vi "Dresden R2R Sputter 03.02.2018 IY24.vi"() -> ()   [LabVIEW 2009] (continued)
                                n21135 = local write "Semi"(TRUE ("Semi")) -> ()
                                }
                                }
                                n21136 = local read "Ch4_Air_press_di"() -> (w22217:bool)
                                n21137 = case shown="True" w22217 {
                                tunnel: [TRUE FALSE] -> w22220
                                frame #0 {
                                }
                                frame #1 {
                                n21138 = Wait Until Next ms Multiple(millisecond multiple=u32 200) -> ()  [unwired: 1 out]
                                }
                                }
                                n21139 = local read "Semi"() -> (w22219:bool)
                                n21140 = Or(x=w22220, y=w22219) -> (x .or. y?=w22218:bool)
                                }
                              }
                              frame #1 {
                              }
                            }
                          }
                          frame #1 {
                            n21141 = local read "Semi"() -> (w22228:bool)
                            n21142 = case shown="False" w22228 {
                              frame #0 {
                                n21143 = Wait Until Next ms Multiple(millisecond multiple=u32 1000) -> ()  [unwired: 1 out]
                                n21144 = local write "Ch4_PV0"(TRUE ("PA0")) -> ()
                                n21145 = local write "Ch4_PA0"(TRUE ("PA0")) -> ()
                              }
                              frame #1 {
                              }
                            }
                          }
                        }
                      }
                      frame #1 {
                      }
                    }
                  }
                  frame #2 {
                    n21146 = local read "Semi"() -> (w22232:bool)
                    n21147 = case shown="False" w22232 {
                      frame #0 {
                        n21148 = stacked-sequence {
                          frame #0 {
                            n21149 = local read "Semi"() -> (w22233:bool)
                            n21150 = case shown="False" w22233 {
                              frame #0 {
                                n21151 = while {
                                i -> [w22240]
                                stop <- w22236 stop-if-true
                                n21152 = Greater?(x=w22240, y=50) -> (0:w22234:bool)
                                n21153 = case shown="True" w22234 {
                                frame #0 {
                                }
                                frame #1 {
                                n21154 = local write "Error Message"("Start up process cancelled because\nchamber door is open.\nPlease close the door." ("Error Message")) -> ()
                                n21155 = local write "Semi"(TRUE ("Semi")) -> ()
                                }
                                }
                                n21156 = local read "Ch4_Ds_di"() -> (w22235:bool)
                                n21157 = case shown="False" w22235 {
                                tunnel: [TRUE FALSE] -> w22238
                                frame #0 {
                                }
                                frame #1 {
                                n21158 = Wait Until Next ms Multiple(millisecond multiple=u32 200) -> ()  [unwired: 1 out]
                                }
                                }
                                n21159 = local read "Semi"() -> (w22237:bool)
                                n21160 = Or(x=w22238, y=w22237) -> (x .or. y?=w22236:bool)
                                }
                              }
                              frame #1 {
                              }
                            }
                          }
                          frame #1 {
                            n21161 = local read "Semi"() -> (w22246:bool)
                            n21162 = case shown="False" w22246 {
                              frame #0 {
                                n21163 = local write "Ch4_PV1"(TRUE ("PA0")) -> ()
                                n21164 = local write "Ch4_PA1"(TRUE ("PA0")) -> ()
                                n21165 = Wait Until Next ms Multiple(millisecond multiple=u32 1000) -> ()  [unwired: 1 out]
                              }
                              frame #1 {
                              }
                            }
                          }
                        }
                      }
                      frame #1 {
                      }
                    }
                  }
                  frame #3 {
                    n21166 = local read "Semi"() -> (w22250:bool)
                    n21167 = case shown="False" w22250 {
                      frame #0 {
                        n21168 = stacked-sequence {
                          frame #0 {
                            n21169 = local read "Semi"() -> (w22251:bool)
                            n21170 = case shown="False" w22251 {
                              frame #0 {
                                n21171 = while {
                                i -> [w22258]
                                stop <- w22254 stop-if-true
                                n21172 = Greater?(x=w22258, y=50) -> (0:w22252:bool)
                                n21173 = case shown="True" w22252 {
                                frame #0 {
                                }
                                frame #1 {
                                n21174 = local write "Error Message"("Start up process cancelled because\nsystem water flow is not enough.\nPlease check main water flow connections." ("Error Message")) -> ()
                                n21175 = local write "Semi"(TRUE ("Semi")) -> ()
                                }
                                }
                                n21176 = local read "Cnt_wfs_di"() -> (w22253:bool)
                                n21177 = case shown="False" w22253 {
                                tunnel: [TRUE FALSE] -> w22256
                                frame #0 {
                                }
                                frame #1 {
                                n21178 = Wait Until Next ms Multiple(millisecond multiple=u32 200) -> ()  [unwired: 1 out]
                                }
                                }
                                n21179 = local read "Semi"() -> (w22255:bool)
                                n21180 = Or(x=w22256, y=w22255) -> (x .or. y?=w22254:bool)
                                }
                              }
                              frame #1 {
                              }
                            }
                          }
                          frame #1 {
                            n21181 = local read "Semi"() -> (w22264:bool)
                            n21182 = case shown="False" w22264 {
                              frame #0 {
                                n21183 = Wait Until Next ms Multiple(millisecond multiple=u32 1000) -> ()  [unwired: 1 out]
                                n21184 = local write "Ch4_PA2"(TRUE ("PA0")) -> ()
                                n21185 = local write "Ch4_PV2"(TRUE ("PA0")) -> ()
                              }
                              frame #1 {
                              }
                            }
                          }
                        }
                      }
                      frame #1 {
                      }
                    }
                  }
                  frame #4 {
                    n21186 = local read "Semi"() -> (w22268:bool)
                    n21187 = case shown="False" w22268 {
                      frame #0 {
                        n21188 = disable-structure shown="Disabled" {
                          frame #0 {
                            n21189 = stacked-sequence {
                              frame #0 {
                                n21190 = local read "Semi"() -> (w22269:bool)
                                n21191 = case shown="False" w22269 {
                                frame #0 {
                                n21192 = local write "Ch4_WFC_do"(TRUE ("Ch1_WFC_do")) -> ()
                                }
                                frame #1 {
                                }
                                }
                              }
                              frame #1 {
                                n21193 = local read "Semi"() -> (w22271:bool)
                                n21194 = case shown="False" w22271 {
                                frame #0 {
                                n21195 = while {
                                i -> [w22278]
                                stop <- w22274 stop-if-true
                                n21196 = Greater?(x=w22278, y=50) -> (0:w22272:bool)
                                n21197 = case shown="True" w22272 {
                                frame #0 {
                                }
                                frame #1 {
                                n21198 = local write "Error Message"("Start up process cancelled because\nchamber water flow is not enough.\nPlease check chamber water \nflow connections." ("Error Message")) -> ()
                                n21199 = local write "Semi"(TRUE ("Semi")) -> ()
                                }
                                }
                                n21200 = local read "Ch4_WFS_di"() -> (w22273:bool)
                                n21201 = case shown="False" w22273 {
                                tunnel: [TRUE FALSE] -> w22276
                                frame #0 {
                                }
                                frame #1 {
                                n21202 = Wait Until Next ms Multiple(millisecond multiple=u32 200) -> ()  [unwired: 1 out]
                                n21203 = local write "Ch4_WFC_do"(TRUE ("Ch1_WFC_do")) -> ()
                                }
                                }
                                n21204 = local read "Semi"() -> (w22275:bool)
                                n21205 = Or(x=w22276, y=w22275) -> (x .or. y?=w22274:bool)
                                }
                                }
                                frame #1 {
                                }
                                }
                              }
                              frame #2 {
                                n21206 = local read "Semi"() -> (w22285:bool)
                                n21207 = case shown="False" w22285 {
                                frame #0 {
                                n21208 = Wait Until Next ms Multiple(millisecond multiple=u32 1000) -> ()  [unwired: 1 out]
                                }
                                frame #1 {
                                }
                                }
                              }
                            }
                          }
                          frame #1 {
                          }
                        }
                      }
                      frame #1 {
                      }
                    }
                  }
                  frame #5 {
                    n21209 = local read "Semi"() -> (w22287:bool)
                    n21210 = case shown="False" w22287 {
                      frame #0 {
                        n21211 = stacked-sequence {
                          frame #0 {
                            n21212 = local read "Semi"() -> (w22288:bool)
                            n21213 = case shown="False" w22288 {
                              frame #0 {
                                n21214 = local write "Ch3_Trns_gv_close_do"(TRUE ("Ch1_WFC_do")) -> ()
                              }
                              frame #1 {
                              }
                            }
                          }
                          frame #1 {
                            n21215 = local read "Semi"() -> (w22290:bool)
                            n21216 = case shown="False" w22290 {
                              frame #0 {
                                n21217 = while {
                                i -> [w22297]
                                stop <- w22293 stop-if-true
                                n21218 = Greater?(x=w22297, y=300) -> (0:w22291:bool)
                                n21219 = case shown="True" w22291 {
                                frame #0 {
                                }
                                frame #1 {
                                n21220 = local write "Error Message"("Start up process cancelled because\nchamber Trns GV between \nCH3 and CH4 not closed.\nPlease check  GV connection." ("Error Message")) -> ()
                                n21221 = local write "Semi"(TRUE ("Semi")) -> ()
                                }
                                }
                                n21222 = local read "Ch3_Trns_gv_close_di"() -> (w22292:bool)
                                n21223 = case shown="False" w22292 {
                                tunnel: [TRUE FALSE] -> w22295
                                frame #0 {
                                }
                                frame #1 {
                                n21224 = Wait Until Next ms Multiple(millisecond multiple=u32 200) -> ()  [unwired: 1 out]
                                n21225 = local write "Ch3_Trns_gv_open_do"(FALSE ("Ch1_Trns_gv_open_do")) -> ()
                                n21226 = local write "Ch3_Trns_gv_close_do"(TRUE ("Ch1_Trns_gv_close_do")) -> ()
                                }
                                }
                                n21227 = local read "Semi"() -> (w22294:bool)
                                n21228 = Or(x=w22295, y=w22294) -> (x .or. y?=w22293:bool)
                                }
                              }
                              frame #1 {
                              }
                            }
                          }
                          frame #2 {
                            n21229 = local read "Semi"() -> (w22305:bool)
                            n21230 = case shown="False" w22305 {
                              frame #0 {
                                w22306 = TRUE ("PA0")
                                n21231 = Wait Until Next ms Multiple(millisecond multiple=u32 1000) -> ()  [unwired: 1 out]
                                n21232 = local write "Ch4_PA4"(w22306) -> ()
                                n21233 = local write "Ch4_PV4"(w22306) -> ()
                              }
                              frame #1 {
                              }
                            }
                          }
                        }
                      }
                      frame #1 {
                      }
                    }
                  }
                }
              }
              frame #1 {
              }
            }
          }
          frame #1 {
            # "ROUTINE CHECK"
            n21234 = local read "Semi"() -> (w22308:bool)
            n21235 = case shown="False" w22308 {
              frame #0 {
                n21236 = local read "Ch4_pressure2"() -> (w22310:dbl)
                n21237 = Greater Or Equal?(x=w22310, y=0.9) -> (x >= y?=w22309:bool)
                n21238 = case shown="True" w22309 {
                  frame #0 {
                    # "PUMPING CH1 LOWER THAN 0.9 TORR"
                    n21239 = local read "Semi"() -> (w22312:bool)
                    n21240 = case shown="False" w22312 {
                      frame #0 {
                        n21241 = stacked-sequence {
                          frame #0 {
                            # "Close CH-VBV"
                            n21242 = local read "Semi"() -> (w22313:bool)
                            n21243 = case shown="False" w22313 {
                              frame #0 {
                                n21244 = stacked-sequence {
                                frame #0 {
                                n21245 = local read "Semi"() -> (w22314:bool)
                                n21246 = case shown="False" w22314 {
                                frame #0 {
                                n21247 = while {
                                i -> [w22321]
                                stop <- w22315 stop-if-true
                                n21248 = Greater?(x=w22321, y=50) -> (0:w22319:bool)
                                n21249 = case shown="True" w22319 {
                                frame #0 {
                                }
                                frame #1 {
                                n21250 = local write "Semi"(TRUE ("Semi")) -> ()
                                n21251 = local write "Error Message"("Start up process  cancelled\nbecause  CH-VBV not closed.\nPlease check  CH4-VBV connections." ("Error Message")) -> ()
                                }
                                }
                                n21252 = local read "Ch4_Ch_vbv_di"() -> (w22318:bool)
                                n21253 = case shown="True" w22318 {
                                tunnel: [TRUE FALSE] -> w22317
                                frame #0 {
                                }
                                frame #1 {
                                n21254 = Wait Until Next ms Multiple(millisecond multiple=u32 200) -> ()  [unwired: 1 out]
                                n21255 = local write "Ch4_Ch_vbv_do"(FALSE ("Ch1_Tp_bv_do")) -> ()
                                }
                                }
                                n21256 = local read "Semi"() -> (w22316:bool)
                                n21257 = Or(x=w22317, y=w22316) -> (x .or. y?=w22315:bool)
                                }
                                }
                                frame #1 {
                                }
                                }
                                }
                                frame #1 {
                                n21258 = local read "Semi"() -> (w22328:bool)
                                n21259 = case shown="False" w22328 {
                                frame #0 {
                                n21260 = local write "Ch4_PV5"(TRUE ("Pd5")) -> ()
                                n21261 = Wait Until Next ms Multiple(millisecond multiple=u32 1000) -> ()  [unwired: 1 out]
                                }
                                frame #1 {
                                }
                                }
                                }
                                }
                              }
                              frame #1 {
                              }
                            }
                          }
                          frame #1 {
                            # "Close PL-VBV"
                            n21262 = local read "Semi"() -> (w22331:bool)
                            n21263 = case shown="False" w22331 {
                              frame #0 {
                                n21264 = stacked-sequence {
                                frame #0 {
                                n21265 = local read "Semi"() -> (w22332:bool)
                                n21266 = case shown="False" w22332 {
                                frame #0 {
                                n21267 = while {
                                i -> [w22339]
                                stop <- w22333 stop-if-true
                                n21268 = Greater?(x=w22339, y=50) -> (0:w22337:bool)
                                n21269 = case shown="True" w22337 {
                                frame #0 {
                                }
                                frame #1 {
                                n21270 = local write "Semi"(TRUE ("Semi")) -> ()
                                n21271 = local write "Error Message"("Start up process  cancelled\nbecause  PL-VBV not closed.\nPlease check PL4-VBV connections." ("Error Message")) -> ()
                                }
                                }
                                n21272 = local read "Ch4_Pl_vbv_di"() -> (w22336:bool)
                                n21273 = case shown="True" w22336 {
                                tunnel: [TRUE FALSE] -> w22335
                                frame #0 {
                                }
                                frame #1 {
                                n21274 = Wait Until Next ms Multiple(millisecond multiple=u32 200) -> ()  [unwired: 1 out]
                                n21275 = local write "Ch4_Pl_vbv_do"(FALSE ("Ch1_Tp_bv_do")) -> ()
                                }
                                }
                                n21276 = local read "Semi"() -> (w22334:bool)
                                n21277 = Or(x=w22335, y=w22334) -> (x .or. y?=w22333:bool)
                                }
                                }
                                frame #1 {
                                }
                                }
                                }
                                frame #1 {
                                n21278 = local read "Semi"() -> (w22346:bool)
                                n21279 = case shown="False" w22346 {
                                frame #0 {
                                n21280 = local write "Ch4_PV6"(TRUE ("P03")) -> ()
                                n21281 = Wait Until Next ms Multiple(millisecond multiple=u32 1000) -> ()  [unwired: 1 out]
                                }
                                frame #1 {
                                }
                                }
                                }
                                }
                              }
                              frame #1 {
                              }
                            }
                          }
                          frame #2 {
                            # "Close CH-ATM"
                            n21282 = local read "Semi"() -> (w22349:bool)
                            n21283 = case shown="False" w22349 {
                              frame #0 {
                                n21284 = stacked-sequence {
                                frame #0 {
                                n21285 = local read "Semi"() -> (w22350:bool)
                                n21286 = case shown="False" w22350 {
                                frame #0 {
                                n21287 = while {
                                i -> [w22357]
                                stop <- w22351 stop-if-true
                                n21288 = Greater?(x=w22357, y=50) -> (0:w22355:bool)
                                n21289 = case shown="True" w22355 {
                                frame #0 {
                                }
                                frame #1 {
                                n21290 = local write "Semi"(TRUE ("Semi")) -> ()
                                n21291 = local write "Error Message"("Start up process  cancelled\nbecause CH-ATM not closed.\nPlease check CH4-ATM connections." ("Error Message")) -> ()
                                }
                                }
                                n21292 = local read "Ch4_Ch_atm_di"() -> (w22354:bool)
                                n21293 = case shown="True" w22354 {
                                tunnel: [TRUE FALSE] -> w22353
                                frame #0 {
                                }
                                frame #1 {
                                n21294 = Wait Until Next ms Multiple(millisecond multiple=u32 200) -> ()  [unwired: 1 out]
                                n21295 = local write "Ch4_Ch_atm_do"(TRUE ("Ch1_Tp_bv_do")) -> ()
                                }
                                }
                                n21296 = local read "Semi"() -> (w22352:bool)
                                n21297 = Or(x=w22353, y=w22352) -> (x .or. y?=w22351:bool)
                                }
                                }
                                frame #1 {
                                }
                                }
                                }
                                frame #1 {
                                n21298 = local read "Semi"() -> (w22364:bool)
                                n21299 = case shown="False" w22364 {
                                frame #0 {
                                n21300 = Wait Until Next ms Multiple(millisecond multiple=u32 1000) -> ()  [unwired: 1 out]
                                n21301 = local write "Ch4_PV7"(TRUE ("P03")) -> ()
                                }
                                frame #1 {
                                }
                                }
                                }
                                }
                              }
                              frame #1 {
                              }
                            }
                          }
                          frame #3 {
                            # "Close PL-ATM"
                            n21302 = local read "Semi"() -> (w22367:bool)
                            n21303 = case shown="False" w22367 {
                              frame #0 {
                                n21304 = stacked-sequence {
                                frame #0 {
                                n21305 = local read "Semi"() -> (w22368:bool)
                                n21306 = case shown="False" w22368 {
                                frame #0 {
                                n21307 = while {
                                i -> [w22375]
                                stop <- w22369 stop-if-true
                                n21308 = Greater?(x=w22375, y=50) -> (0:w22373:bool)
                                n21309 = case shown="True" w22373 {
                                frame #0 {
                                }
                                frame #1 {
                                n21310 = local write "Semi"(TRUE ("Semi")) -> ()
                                n21311 = local write "Error Message"("Start up process  cancelled\nbecause PL-ATM not closed.\nPlease check PL4-ATM connections." ("Error Message")) -> ()
                                }
                                }
                                n21312 = local read "Ch4_Pl_atm_di"() -> (w22372:bool)
                                n21313 = case shown="True" w22372 {
                                tunnel: [TRUE FALSE] -> w22371
                                frame #0 {
                                }
                                frame #1 {
                                n21314 = Wait Until Next ms Multiple(millisecond multiple=u32 200) -> ()  [unwired: 1 out]
                                n21315 = local write "Ch4_Pl_atm_do"(TRUE ("Ch1_Tp_bv_do")) -> ()
                                }
                                }
                                n21316 = local read "Semi"() -> (w22370:bool)
                                n21317 = Or(x=w22371, y=w22370) -> (x .or. y?=w22369:bool)
                                }
                                }
                                frame #1 {
                                }
                                }
                                }
                                frame #1 {
                                n21318 = local read "Semi"() -> (w22382:bool)
                                n21319 = case shown="False" w22382 {
                                frame #0 {
                                n21320 = Wait Until Next ms Multiple(millisecond multiple=u32 1000) -> ()  [unwired: 1 out]
                                n21321 = local write "Ch4_PV8"(TRUE ("P03")) -> ()
                                }
                                frame #1 {
                                }
                                }
                                }
                                }
                              }
                              frame #1 {
                              }
                            }
                          }
                          frame #4 {
                            # "START MP"
                            n21322 = local read "Semi"() -> (w22385:bool)
                            n21323 = case shown="False" w22385 {
                              frame #0 {
                                n21324 = stacked-sequence {
                                frame #0 {
                                n21325 = local read "Semi"() -> (w22386:bool)
                                n21326 = case shown="False" w22386 {
                                frame #0 {
                                n21327 = while {
                                i -> [w22393]
                                stop <- w22387 stop-if-true
                                n21328 = Greater?(x=w22393, y=50) -> (0:w22391:bool)
                                n21329 = case shown="True" w22391 {
                                frame #0 {
                                }
                                frame #1 {
                                n21330 = local write "Semi"(TRUE ("Semi")) -> ()
                                n21331 = local write "Error Message"("Start up process  cancelled\nbecause MP4 not started.\nPlease check MP4 connections." ("Error Message")) -> ()
                                }
                                }
                                n21332 = local read "Ch4_Mp_di"() -> (w22390:bool)
                                n21333 = case shown="False" w22390 {
                                tunnel: [FALSE TRUE] -> w22389
                                frame #0 {
                                n21334 = Wait Until Next ms Multiple(millisecond multiple=u32 200) -> ()  [unwired: 1 out]
                                n21335 = local write "Ch4_Mp_do"(TRUE ("Ch1_Tp_bv_do")) -> ()
                                }
                                frame #1 {
                                }
                                }
                                n21336 = local read "Semi"() -> (w22388:bool)
                                n21337 = Or(x=w22389, y=w22388) -> (x .or. y?=w22387:bool)
                                }
                                }
                                frame #1 {
                                }
                                }
                                }
                                frame #1 {
                                n21338 = local read "Semi"() -> (w22400:bool)
                                n21339 = case shown="False" w22400 {
                                frame #0 {
                                n21340 = local write "Ch4_PV9"(TRUE ("P03")) -> ()
                                n21341 = Wait Until Next ms Multiple(millisecond multiple=u32 1000) -> ()  [unwired: 1 out]
                                }
                                frame #1 {
                                }
                                }
                                }
                                }
                              }
                              frame #1 {
                              }
                            }
                          }
                          frame #5 {
                            # "CHECK PL-PRESSURE"
                            n21342 = local read "Semi"() -> (w22403:bool)
                            n21343 = case shown="False" w22403 {
                              frame #0 {
                                n21344 = stacked-sequence {
                                frame #0 {
                                n21345 = local read "Semi"() -> (w22404:bool)
                                n21346 = case shown="False" w22404 {
                                frame #0 {
                                n21347 = while {
                                i -> [w22413]
                                stop <- w22408 stop-if-true
                                n21348 = Greater?(x=w22413, y=240) -> (0:w22411:bool)
                                n21349 = case shown="True" w22411 {
                                frame #0 {
                                }
                                frame #1 {
                                n21350 = local write "Semi"(TRUE ("Semi")) -> ()
                                n21351 = local write "Error Message"("Start up process was cancelled.\nPlease check Pipeline \nvacuum connections." ("Error Message")) -> ()
                                }
                                }
                                n21352 = local read "Pl_pg_press_ch4"() -> (w22407:dbl)
                                n21353 = Less?(x=w22407, y=0.9) -> (x < y?=w22405:bool)
                                n21354 = case shown="False" w22405 {
                                tunnel: [FALSE TRUE] -> w22410
                                frame #0 {
                                n21355 = Wait Until Next ms Multiple(millisecond multiple=u32 200) -> ()  [unwired: 1 out]
                                }
                                frame #1 {
                                }
                                }
                                n21356 = local read "Semi"() -> (w22409:bool)
                                n21357 = Or(x=w22410, y=w22409) -> (x .or. y?=w22408:bool)
                                }
                                }
                                frame #1 {
                                }
                                }
                                }
                                frame #1 {
                                n21358 = local read "Semi"() -> (w22419:bool)
                                n21359 = case shown="False" w22419 {
                                frame #0 {
                                n21360 = Wait Until Next ms Multiple(millisecond multiple=u32 1000) -> ()  [unwired: 1 out]
                                n21361 = local write "Ch4_PV10"(TRUE ("P03")) -> ()
                                }
                                frame #1 {
                                }
                                }
                                }
                                }
                              }
                              frame #1 {
                              }
                            }
                          }
                          frame #6 {
                            # "CHECK CH-PRESSURE"
                            n21362 = local read "Semi"() -> (w22422:bool)
                            n21363 = case shown="False" w22422 {
                              frame #0 {
                                n21364 = stacked-sequence {
                                frame #0 {
                                n21365 = local read "Semi"() -> (w22423:bool)
                                n21366 = case shown="False" w22423 {
                                frame #0 {
                                n21367 = while {
                                i -> [w22432]
                                stop <- w22427 stop-if-true
                                n21368 = Greater?(x=w22432, y=50) -> (0:w22430:bool)
                                n21369 = case shown="True" w22430 {
                                frame #0 {
                                }
                                frame #1 {
                                n21370 = local write "Semi"(TRUE ("Semi")) -> ()
                                n21371 = local write "Error Message"("Start up process was cancelled.\nPlease check chamber \nvacuum connections." ("Error Message")) -> ()
                                }
                                }
                                n21372 = local read "Ch4pressure"() -> (w22426:dbl)
                                n21373 = Less?(x=w22426, y=0.9) -> (x < y?=w22424:bool)
                                n21374 = case shown="False" w22424 {
                                tunnel: [FALSE TRUE] -> w22429
                                frame #0 {
                                n21375 = Wait Until Next ms Multiple(millisecond multiple=u32 200) -> ()  [unwired: 1 out]
                                }
                                frame #1 {
                                }
                                }
                                n21376 = local read "Semi"() -> (w22428:bool)
                                n21377 = Or(x=w22429, y=w22428) -> (x .or. y?=w22427:bool)
                                }
                                }
                                frame #1 {
                                }
                                }
                                }
                                frame #1 {
                                n21378 = local read "Semi"() -> (w22438:bool)
                                n21379 = case shown="False" w22438 {
                                frame #0 {
                                n21380 = Wait Until Next ms Multiple(millisecond multiple=u32 1000) -> ()  [unwired: 1 out]
                                n21381 = local write "Ch4_PV11"(TRUE ("P03")) -> ()
                                }
                                frame #1 {
                                }
                                }
                                }
                                }
                              }
                              frame #1 {
                              }
                            }
                          }
                          frame #7 {
                            # "OPEN TP-BV"
                            n21382 = local read "Semi"() -> (w22441:bool)
                            n21383 = case shown="False" w22441 {
                              frame #0 {
                                n21384 = stacked-sequence {
                                frame #0 {
                                n21385 = local read "Semi"() -> (w22442:bool)
                                n21386 = case shown="False" w22442 {
                                frame #0 {
                                n21387 = while {
                                i -> [w22449]
                                stop <- w22444 stop-if-true
                                n21388 = Greater?(x=w22449, y=50) -> (0:w22447:bool)
                                n21389 = case shown="True" w22447 {
                                frame #0 {
                                }
                                frame #1 {
                                n21390 = local write "Semi"(TRUE ("Semi")) -> ()
                                n21391 = local write "Error Message"("Start up process  cancelled\nbecause  TP-BV not opened.\nPlease check TP-BV4 connections." ("Error Message")) -> ()
                                }
                                }
                                n21392 = local read "Ch4_Tp_bv_di"() -> (w22443:bool)
                                n21393 = case shown="False" w22443 {
                                tunnel: [FALSE TRUE] -> w22446
                                frame #0 {
                                n21394 = Wait Until Next ms Multiple(millisecond multiple=u32 200) -> ()  [unwired: 1 out]
                                n21395 = local write "Ch4_Tp_bv_do"(TRUE ("Ch1_Tp_bv_do")) -> ()
                                }
                                frame #1 {
                                }
                                }
                                n21396 = local read "Semi"() -> (w22445:bool)
                                n21397 = Or(x=w22446, y=w22445) -> (x .or. y?=w22444:bool)
                                }
                                }
                                frame #1 {
                                }
                                }
                                }
                                frame #1 {
                                n21398 = local read "Semi"() -> (w22456:bool)
                                n21399 = case shown="False" w22456 {
                                frame #0 {
                                n21400 = local write "Ch4_PV12"(TRUE ("P03")) -> ()
                                n21401 = Wait Until Next ms Multiple(millisecond multiple=u32 1000) -> ()  [unwired: 1 out]
                                }
                                frame #1 {
                                }
                                }
                                }
                                }
                              }
                              frame #1 {
                              }
                            }
                          }
                          frame #8 {
                            # "OPEN PC-BV"
                            n21402 = local read "Semi"() -> (w22459:bool)
                            n21403 = case shown="False" w22459 {
                              frame #0 {
                                n21404 = stacked-sequence {
                                frame #0 {
                                n21405 = local read "Semi"() -> (w22460:bool)
                                n21406 = case shown="False" w22460 {
                                frame #0 {
                                n21407 = stacked-sequence {
                                frame #0 {
                                n21408 = local read "Semi"() -> (w22461:bool)
                                n21409 = case shown="False" w22461 {
                                frame #0 {
                                n21410 = local write "Pc_bv4_auto_open"(TRUE ("Tp1_auto_start")) -> ()
                                }
                                frame #1 {
                                }
                                }
                                }
                                frame #1 {
                                n21411 = local read "Semi"() -> (w22463:bool)
                                n21412 = case shown="False" w22463 {
                                frame #0 {
                                n21413 = Wait (ms)(milliseconds to wait=u32 1000) -> ()  [unwired: 1 out]
                                }
                                frame #1 {
                                }
                                }
                                }
                                frame #2 {
                                n21414 = local read "Semi"() -> (w22465:bool)
                                n21415 = case shown="False" w22465 {
                                frame #0 {
                                n21416 = while {
                                i -> [w22471]
                                stop <- w22467 stop-if-true
                                n21417 = local read "Pc_bv_opened_ch4"() -> (w22469:bool)
                                n21418 = Greater?(x=w22471, y=120) -> (0:w22470:bool)
                                n21419 = local read "Semi"() -> (w22468:bool)
                                n21420 = Compound Arithmetic op=OR(w22468, w22469, w22470) -> (w22467:bool)
                                n21421 = Wait (ms)(milliseconds to wait=u32 500) -> ()  [unwired: 1 out]
                                }
                                }
                                frame #1 {
                                }
                                }
                                }
                                frame #3 {
                                n21422 = local read "Semi"() -> (w22473:bool)
                                n21423 = case shown="False" w22473 {
                                frame #0 {
                                n21424 = local read "Pc_bv_opened_ch4"() -> (w22474:bool)
                                n21425 = case shown="False" w22474 {
                                frame #0 {
                                n21426 = local write "Pc_bv4_auto_open"(TRUE ("Pc_bv1_auto_open")) -> ()
                                }
                                frame #1 {
                                }
                                }
                                }
                                frame #1 {
                                }
                                }
                                }
                                frame #4 {
                                n21427 = local read "Semi"() -> (w22476:bool)
                                n21428 = case shown="False" w22476 {
                                frame #0 {
                                n21429 = local read "Pc_bv_opened_ch4"() -> (w22477:bool)
                                n21430 = case shown="False" w22477 {
                                frame #0 {
                                n21431 = Wait (ms)(milliseconds to wait=u32 1000) -> ()  [unwired: 1 out]